vi "FlexMag - 23-03-2023.vi"() -> ()   [LabVIEW 2018]
uses:
  <vilib>/Instr/_visa.llb/VISA Configure Serial Port (Instr).vi
  nimodbus121/71/vi.lib/NI Modbus.llb/MB Serial Master Query Write Single Coil (poly).vi
  <vilib>/picture/picture.llb/Draw True-Color Pixmap.vi
  <vilib>/Utility/file.llb/Read Delimited Spreadsheet (string).vi
  <vilib>/addons/control/pid/pid.llb/PID (DBL).vi
  <vilib>/addons/control/pid/NI_PID_pid.lvlib
panel:
  in  "initial cover tab":enum32{"Page 1"}(tab)
  out "initial string":string
  out "Slide":u8(slide) scale=0.0..100.0
  out "MAG gui":bool
  in  "buzzer off":bool
  in  "ABORT":bool
  out "Description":string
  out "Warning Message":string
  in  "clear warning":bool
  out "System Status":string
  in  "Recipe Tab":enum32{"Page 1", "Page 2", "Page 3"}(tab)
  in  "R Recipe Selection":u16(ring) items=["single recipe", "multilayer recipe"]
  in  "R Web Selection":u16(ring) items=["web", "other"]
  in  "R tension value":dbl=8.0
  in  "R web speed":dbl=250.0
  in  "R web thickness":dbl=50.0
  in  "R left initial diameter":dbl
  in  "R core diameter":dbl=93.0
  in  "R Ar set sccm":dbl=20.0
  in  "R Pressure set mbar":dbl=0.005 format="%#_1e"
  in  "R DC Sputter Chamber Selection":enum32{"chamber II", "chamber III"}(radio)
  in  "R single process selection":enum32{"microwave", "dcsputter", "rfsputter"}(radio)
  in  "R Substrate Material":string
  in  "R Recipe Name":string
  in  "load recipe from path":bool
  out "path for loading recipe":path
  out "process file list 2":string
  out "L dc step numbers":string
  out "L rf step numbers":string
  out "L pressure":string
  out "L argon flow":string
  out "L rf length step 10":string
  out "L rf length step 9":string
  out "L rf length step 8":string
  out "L rf length step 7":string
  out "L rf length step 6":string
  out "L rf length step 5":string
  out "L rf length step 4":string
  out "L rf length step 3":string
  out "L rf length step 2":string
  out "L rf length step 1":string
  out "L rf power step 10":string
  out "L rf power step 9":string
  out "L rf power step 8":string
  out "L rf power step 7":string
  out "L rf power step 6":string
  out "L rf power step 5":string
  out "L rf power step 4":string
  out "L rf power step 3":string
  out "L rf power step 2":string
  out "L rf power step 1":string
  out "L dc length step 10":string
  out "L dc length step 9":string
  out "L dc length step 8":string
  out "L dc length step 7":string
  out "L dc length step 6":string
  out "L dc length step 5":string
  out "L dc length step 4":string
  out "L dc length step 3":string
  out "L dc length step 2":string
  out "L dc length step 1":string
  out "L dc power step 10":string
  out "L dc power step 9":string
  out "L dc power step 8":string
  out "L dc power step 7":string
  out "L dc power step 6":string
  out "L dc power step 5":string
  out "L dc power step 4":string
  out "L dc power step 3":string
  out "L dc power step 2":string
  out "L dc power step 1":string
  out "L microwave power":string
  out "L chamber selection":string
  out "L single process type selection":string
  out "L tension  value":string
  out "L web speed":string
  out "L web thickness":string
  out "L left init diamater":string
  out "L core diamater":string
  out "L web selection":string
  out "L recipe selection":string
  out "L sbs name":string
  out "L recipe name":string
  out "L dc power step 11":string
  out "L dc power step 12":string
  out "L dc power step 13":string
  out "L dc power step 14":string
  out "L dc power step 15":string
  out "L dc power step 16":string
  out "L dc power step 17":string
  out "L dc power step 18":string
  out "L dc power step 19":string
  out "L dc power step 20":string
  out "L dc length step 11":string
  out "L dc length step 12":string
  out "L dc length step 13":string
  out "L dc length step 14":string
  out "L dc length step 15":string
  out "L dc length step 16":string
  out "L dc length step 17":string
  out "L dc length step 18":string
  out "L dc length step 19":string
  out "L dc length step 20":string
  out "L rf power step 11":string
  out "L rf power step 12":string
  out "L rf power step 13":string
  out "L rf power step 14":string
  out "L rf power step 15":string
  out "L rf power step 16":string
  out "L rf power step 17":string
  out "L rf power step 18":string
  out "L rf power step 19":string
  out "L rf power step 20":string
  out "L rf length step 11":string
  out "L rf length step 12":string
  out "L rf length step 13":string
  out "L rf length step 14":string
  out "L rf length step 15":string
  out "L rf length step 16":string
  out "L rf length step 17":string
  out "L rf length step 18":string
  out "L rf length step 19":string
  out "L rf length step 20":string
  in  "R DC number steps":dbl
  in  "R rf step length 1":dbl
  in  "R rf step length 2":dbl
  in  "R rf step length 3":dbl
  in  "R rf step length 4":dbl
  in  "R rf step length 6":dbl
  in  "R rf step length 7":dbl
  in  "R rf step length 8":dbl
  in  "R rf step length 9":dbl
  in  "R rf step length 5":dbl
  in  "R rf step length 10":dbl
  in  "R dc step power 1":dbl
  in  "R dc step power 2":dbl
  in  "R dc step power 3":dbl
  in  "R dc step power 4":dbl
  in  "R dc step power 6":dbl
  in  "R dc step power 7":dbl
  in  "R dc step power 8":dbl
  in  "R dc step power 9":dbl
  in  "R dc step power 5":dbl
  in  "R dc step power 10":dbl
  in  "R dc step length 1":dbl
  in  "R dc step length 2":dbl
  in  "R dc step length 3":dbl
  in  "R dc step length 4":dbl
  in  "R dc step length 6":dbl
  in  "R dc step length 7":dbl
  in  "R dc step length 8":dbl
  in  "R dc step length 9":dbl
  in  "R dc step length 5":dbl
  in  "R dc step length 10":dbl
  in  "R rf step power 1":dbl
  in  "R rf step power 2":dbl
  in  "R rf step power 3":dbl
  in  "R rf step power 4":dbl
  in  "R rf step power 8":dbl
  in  "R rf step power 5":dbl
  in  "R rf step power 6":dbl
  in  "R rf step power 9":dbl
  in  "R rf step power 7":dbl
  in  "R rf step power 10":dbl
  in  "R power microwave":dbl
  in  "R RF number steps":dbl
  in  "R dc step power 11":dbl
  in  "R dc step power 12":dbl
  in  "R dc step power 13":dbl
  in  "R dc step power 14":dbl
  in  "R dc step power 15":dbl
  in  "R dc step power 16":dbl
  in  "R dc step power 17":dbl
  in  "R dc step power 18":dbl
  in  "R dc step power 19":dbl
  in  "R dc step power 20":dbl
  in  "R dc step length 11":dbl
  in  "R dc step length 12":dbl
  in  "R dc step length 13":dbl
  in  "R dc step length 14":dbl
  in  "R dc step length 15":dbl
  in  "R dc step length 16":dbl
  in  "R dc step length 17":dbl
  in  "R dc step length 18":dbl
  in  "R dc step length 19":dbl
  in  "R dc step length 20":dbl
  in  "GUI_Tab":T1(tab)
  in  "Tab Pressure Graph":enum32{"CH 1", "CH 2", "CH 3", "CH 4"}(tab)
  out "CH 1 Pressure":dbl(graph)
  out "CH 2 Pressure":dbl(graph)
  out "CH 3 Pressure":dbl(graph)
  out "CH 4 Pressure":dbl(graph)
  in  "pid graph":enum32{"Page 1"}(tab)
  out "Waveform Chart":dbl(graph)
  in  "cc3 timer tab":enum32{"Page 1"}(tab)
  in  "cc3 open gui":bool
  in  "cc3 close gui":bool
  in  "cc1 timer tab":enum32{"Page 1"}(tab)
  in  "cc1 close gui":bool
  in  "cc1 open gui":bool
  in  "cc2 timer tab":enum32{"Page 1"}(tab)
  in  "cc2 open gui":bool
  in  "cc2 close gui":bool
  in  "cc4 timer tab":enum32{"Page 1"}(tab)
  in  "cc4 open gui":bool
  in  "cc4 close gui":bool
  in  "bgbv2 timer tab":enum32{"Page 1"}(tab)
  in  "bgbv2 open gui":bool
  in  "bgbv2 close gui":bool
  in  "bgbv3 timer tab":enum32{"Page 1"}(tab)
  in  "bgbv3 open gui":bool
  in  "bgbv3 close gui":bool
  in  "bgbv1 timer tab":enum32{"Page 1"}(tab)
  in  "bgbv1 close gui":bool
  in  "bgbv1 open gui":bool
  in  "bgbv4 timer tab":enum32{"Page 1"}(tab)
  in  "bgbv4 open gui":bool
  in  "bgbv4 close gui":bool
  in  "tp1 timer tab":enum32{"Page 1"}(tab)
  in  "Tp1 stop gui":bool
  in  "Tp1 start gui":bool
  out "ch1_2 vacuum level":string
  out "ch2_3 vacuum level":string
  out "ch3_4 vacuum level":string
  in  "CH3-4 trnsgv timer tab":enum32{"Page 1"}(tab)
  in  "CH3-4 trns open gui":bool
  in  "CH3-4 trns close gui":bool
  in  "CH2-3 trnsgv timer tab":enum32{"Page 1"}(tab)
  in  "CH2-3 trns open gui":bool
  in  "CH2-3 trns close gui":bool
  in  "CH1-2 trnsgv timer tab":enum32{"Page 1"}(tab)
  in  "CH1-2 trns open gui":bool
  in  "CH1-2 trns close gui":bool
  in  "ch4 trnsbp right timer tab":enum32{"Page 1"}(tab)
  in  "ch4 trnsbp right close gui":bool
  in  "ch4 trnsbp right open gui":bool
  in  "ch3 trnsbp left timer tab":enum32{"Page 1"}(tab)
  in  "ch3 trnsbp left close gui":bool
  in  "ch3 trnsbp left open gui":bool
  in  "ch3 trnsbp right timer tab":enum32{"Page 1"}(tab)
  in  "ch3 trnsbp right close gui":bool
  in  "ch3 trnsbp right open gui":bool
  in  "ch2 trnsbp left timer tab":enum32{"Page 1"}(tab)
  in  "ch2 trnsbp left close gui":bool
  in  "ch2 trnsbp left open gui":bool
  in  "ch2 trnsbp right timer tab":enum32{"Page 1"}(tab)
  in  "ch2 trnsbp right close gui":bool
  in  "ch2 trnsbp right open gui":bool
  in  "ch1 trnsbp left timer tab":enum32{"Page 1"}(tab)
  in  "ch1 trnsbp left close gui":bool
  in  "ch1 trnsbp left open gui":bool
  out "ch4 ch pg mbar gui":dbl format="%#_2e"
  out "ch4 cc mbar gui":dbl format="%#_2e"
  out "ch4 pl pg mbar gui":dbl format="%#_2e"
  out "ch3 cc mbar gui":dbl format="%#_2e"
  out "ch3 ch pg mbar gui":dbl format="%#_2e"
  out "ch3 pl pg mbar gui":dbl format="%#_2e"
  out "ch2 ch pg mbar gui":dbl format="%#_2e"
  out "ch2 pl pg mbar gui":dbl format="%#_2e"
  out "ch2 cc mbar gui":dbl format="%#_2e"
  out "ch1 cc mbar gui":dbl format="%#_2e"
  out "ch1 ch pg mbar gui":dbl format="%#_2e"
  out "ch1 pl pg mbar gui":dbl format="%#_2e"
  out "Tp1 speed gui":i32
  out "Tp2 speed gui":i32
  out "Tp3 speed gui":i32
  out "Tp4 speed gui":i32
  in  "tp3 timer tab":enum32{"Page 1"}(tab)
  in  "Tp3 stop gui":bool
  in  "Tp3 start gui":bool
  in  "tp4 timer tab":enum32{"Page 1"}(tab)
  in  "Tp4 stop gui":bool
  in  "Tp4 start gui":bool
  in  "tp2 timer tab":enum32{"Page 1"}(tab)
  in  "Tp2 stop gui":bool
  in  "Tp2 start gui":bool
  in  "pcgv4 timer tab":enum32{"Page 1"}(tab)
  in  "pcgv4 open gui":bool
  in  "pcgv4 close gui":bool
  in  "pcgv3 timer tab":enum32{"Page 1"}(tab)
  in  "pcgv3 close gui":bool
  in  "pcgv3 open gui":bool
  in  "pcgv2 timer tab":enum32{"Page 1"}(tab)
  in  "pcgv2 close gui":bool
  in  "pcgv2 open gui":bool
  in  "pcgv1 timer tab":enum32{"Page 1"}(tab)
  in  "pcgv1 close gui":bool
  in  "pcgv1 open gui":bool
  out "Ch1_baratron_pressure_mbar":dbl format="%.1e"
  out "Ch2_baratron_pressure_mbar":dbl format="%.1e"
  out "Ch3_baratron_pressure_mbar":dbl format="%.1e"
  out "Ch4_baratron_pressure_mbar":dbl format="%.1e"
  in  "tpbv3 timer tab":enum32{"Page 1"}(tab)
  in  "tpbv3 open gui":bool
  in  "tpbv3 close gui":bool
  in  "tpbv2 timer tab":enum32{"Page 1"}(tab)
  in  "tpbv2 open gui":bool
  in  "tpbv2 close gui":bool
  in  "tpbv1 timer tab":enum32{"Page 1"}(tab)
  in  "tpbv1 close gui":bool
  in  "tpbv1 open gui":bool
  in  "chvbv4 timer tab":enum32{"Page 1"}(tab)
  in  "chvbv4 open gui":bool
  in  "chvbv4 close gui":bool
  in  "chvbv3 timer tab":enum32{"Page 1"}(tab)
  in  "chvbv3 open gui":bool
  in  "chvbv3 close gui":bool
  in  "chvbv2 timer tab":enum32{"Page 1"}(tab)
  in  "chvbv2 open gui":bool
  in  "chvbv2 close gui":bool
  in  "chvbv1 timer tab":enum32{"Page 1"}(tab)
  in  "chvbv1 close gui":bool
  in  "chvbv1 open gui":bool
  in  "tpbv4 timer tab":enum32{"Page 1"}(tab)
  in  "tpbv4 open gui":bool
  in  "tpbv4 close gui":bool
  in  "plvbv4 timer tab":enum32{"Page 1"}(tab)
  in  "plvbv4 open gui":bool
  in  "plvbv4 close gui":bool
  in  "plvbv3 timer tab":enum32{"Page 1"}(tab)
  in  "plvbv3 open gui":bool
  in  "plvbv3 close gui":bool
  in  "plvbv1 timer tab":enum32{"Page 1"}(tab)
  in  "plvbv1 close gui":bool
  in  "plvbv1 open gui":bool
  in  "plvbv2 timer tab":enum32{"Page 1"}(tab)
  in  "plvbv2 open gui":bool
  in  "plvbv2 close gui":bool
  in  "mp4 timer tab":enum32{"Page 1"}(tab)
  in  "mp4 start gui":bool
  in  "mp4 stop gui":bool
  in  "mp3 timer tab":enum32{"Page 1"}(tab)
  in  "mp3 start gui":bool
  in  "mp3 stop gui":bool
  in  "mp2 timer tab":enum32{"Page 1"}(tab)
  in  "mp2 start gui":bool
  in  "mp2 stop gui":bool
  in  "mp1 timer tab":enum32{"Page 1"}(tab)
  in  "mp1 start gui":bool
  in  "mp1 stop gui":bool
  in  "Tab Control":T2(tab)
  in  "OK Button":bool
  in  "cassette position selection":u16(ring)=1 items=["CH1"=1, "CH2"=2, "CH3"=3, "CH4"=4]
  in  "hide pressure graphs":bool
  in  "show pressure graphs":bool
  in  "graph sec":dbl=3.0
  in  "transfer vacuum":bool
  out "present location":dbl=inf format="%#_2g"
  in  "target chamber":dbl=1.0 min=1.0 max=4.0
  in  "transfer atm":bool
  in  "CHAMBERS CONTROL":T3(tab)
  in  "Tp1 normal speed gui":bool
  in  "Tp1 low speed gui":bool
  in  "Tp1 set speed gui":bool
  in  "Low_speed_value":ext=60.0
  in  "Pump Down CH1":bool
  in  "Shut Down CH1":bool
  in  "ch1 desired pressure":dbl format="%#_2e"
  in  "Low_speed_value 2":ext=60.0
  in  "Tp2 normal speed gui":bool
  in  "Tp2 low speed gui":bool
  in  "Tp2 set speed gui":bool
  in  "Pump Down CH2":bool
  in  "Shut Down CH2":bool
  in  "ch2 desired pressure":dbl format="%#_2e"
  in  "Low_speed_value 3":ext=60.0
  in  "Tp3 normal speed gui":bool
  in  "Tp3 low speed gui":bool
  in  "Tp3 set speed gui":bool
  in  "Pump Down CH3":bool
  in  "Shut Down CH3":bool
  in  "ch3 desired pressure":dbl format="%#_2e"
  in  "Pump Down CH4":bool
  in  "Shut Down CH4":bool
  in  "ch4 desired pressure":dbl=5e-05 format="%#_2e"
  in  "Low_speed_value 4":ext=60.0
  in  "Tp4 normal speed gui":bool
  in  "Tp4 low speed gui":bool
  in  "Tp4 set speed gui":bool
  in  "QR continuous mode gui":bool
  in  "QR off mode gui":bool
  out "qr read statue gui":string
  in  "max rotation number":dbl=300.0
  out "current step":dbl
  in  "step count":dbl
  out "lap number left actual":dbl
  out "lap number right actual":dbl
  in  "tension value":dbl=10.0
  in  "setpoint":dbl=550.0
  out "process variable":dbl
  out "ch4_srv_piston_status":string
  out "ch3_srv_piston_status":string
  out "ch2_srv_piston_status":string
  out "ch1_srv_piston_status":string
  out "ch4_petcool_status":string
  out "ch3_petcool_status":string
  out "ch2_petcool_status":string
  out "ch1_petcool_status":string
  out "ch4_cst_fix_status":string
  out "ch3_cst_fix_status":string
  out "ch2_cst_fix_status":string
  out "ch1_cst_fix_status":string
  in  "forward roll":bool
  in  "back roll":bool
  in  "stop roll":bool
  out "parameters led":bool
  in  "CH1 cstfix up":bool
  in  "CH1 cstfix down":bool
  in  "CH2 cstfix down":bool
  in  "CH2 cstfix up":bool
  in  "CH4 cstfix down":bool
  in  "CH4 cstfix up":bool
  in  "CH3 cstfix down":bool
  in  "CH3 cstfix up":bool
  in  "CH1 petcool down":bool
  in  "CH1 petcool up":bool
  in  "CH2 petcool down":bool
  in  "CH2 petcool up":bool
  in  "CH3 petcool down":bool
  in  "CH3 petcool up":bool
  in  "CH4 petcool down":bool
  in  "CH4 petcool up":bool
  in  "CH4 srv back":bool
  in  "CH4 srv forward":bool
  in  "CH3 srv back":bool
  in  "CH3 srv forward":bool
  in  "CH2 srv back":bool
  in  "CH2 srv forward":bool
  in  "CH1 srv back":bool
  in  "CH1 srv forward":bool
  in  "cycle roll stop":bool
  in  "cycle roll start":bool
  out "Remaining Cycle":u8
  in  "Number of Cycle":u8=10 min=1
  out "rolling direction gui":bool
  in  "load process file":bool
  in  "stop coating":bool
  in  "coating start":bool
  in  "CH1 LN2":bool
  in  "Stop auto LN2":bool
  in  "CH4 LN2":bool
  in  "CH2 LN2":bool
  in  "CH3 LN2":bool
  in  "water bypass":bool=TRUE
  out "process file list":string
  out "current recipe number":i32
  in  "creat recipe file":bool
  in  "creat process file":bool
  in  "Change Rolling Direction":bool
  out "Total Status":string
  out "Total Warning":string
  in  "hide service tab":bool
  in  "show service tab":bool
  in  "service tab":string
  out "ch1_door_open":string
  out "ch2_door_open":string
  out "ch4_door_open":string
  out "ch3_door_open":string
  out "General View":picture
  in  "bgbv4 close gui 2":bool
  in  "bgbv4 open gui 2":bool
  in  "sov4 timer tab":enum32{"Page 1"}(tab)
  in  "sov4 close gui":bool
  in  "sov4 open gui":bool
  out "ch4 ch pg mbar gui 1":dbl format="%#_2e"
  out "ch4 cc mbar gui 1":dbl format="%#_2e"
  out "Ch4_baratron_pressure_mbar 2":dbl format="%.1e"
  out "CH4 front main":picture
  out "CH4 top main":picture
  in  "cc4 close gui 2":bool
  in  "cc4 open gui 2":bool
  in  "Baratron4 set zero gui":bool
  in  "pcgv4 set pressure":bool
  in  "pcgv4 set position gui":bool
  out "pcgv4 position":i32
  in  "pcgv4 set position value":dbl
  in  "pcgv4 set pressure value mbar":dbl=0.005 format="%.1e"
  in  "sov4 close gui 2":bool
  in  "sov4 open gui 2":bool
  out "Ch4_baratron_pressure_mbar 3":dbl format="%.1e"
  in  "Rf_control_tab":T4(tab)
  in  "RF off":bool
  in  "RF on":bool
  in  "RF host":bool
  out "RF Net Power :":u32
  in  "set rf":bool
  in  "RF_forward_power_1":i16
  out "RF Bias:":u32
  in  "Ramp up Time:":dbl
  out "Ramp Up Left Time:":dbl
  in  "Ramp Down Time :":dbl
  out "Ramp Down Left Time:":dbl
  in  "Ramp Up time":bool
  in  "Ramp down time":bool
  out "Pulsing ON/OFF :":bool
  in  "Duty Cycle :":i8
  in  "Frequency :":i64 caption="FREQUENCY"
  in  "set frequency":bool
  in  "set duty":bool
  in  "Pulsing_off":bool
  in  "internal":bool
  in  "Set CL Position:":dbl
  in  "Set CT Position:":dbl
  out "CL Position:":dbl
  out "CT Position:":dbl
  in  "set seri cap pos 2":bool
  in  "set cap pos":bool
  in  "oto tuner":bool
  in  "manuel tuner":bool
  in  "ch4 ar set zero":bool
  in  "ch4 ar set":bool
  out "ch4 argon mfc actual":dbl format="%#.3f"
  in  "ch4 argon mfc set":dbl
  in  "CH3 water close gui":bool
  in  "CH3 water open gui":bool
  in  "bgbv3 open gui 2":bool
  in  "bgbv3 close gui 2":bool
  out "CH3 MAG Active":bool
  in  "ch3 mag active gui":bool
  in  "sov3 timer tab":enum32{"Page 1"}(tab)
  in  "sov3 close gui":bool
  in  "sov3 open gui":bool
  out "ch3 cc mbar gui 1":dbl format="%#_2e"
  out "ch3 ch pg mbar gui 1":dbl format="%#_2e"
  out "Ch3_baratron_pressure_mbar 2":dbl format="%.1e"
  out "CH3 front main":picture
  out "CH3 top main":picture
  in  "cc3 open gui 2":bool
  in  "cc3 close gui 2":bool
  in  "Baratron3 auto set zero":bool
  in  "pcgv3 set pressure gui":bool
  in  "pcgv3 set position":bool
  out "pcgv3 position":i32
  in  "pcgv3 set position value":dbl
  in  "pcgv3 set pressure value mbar":dbl=0.005 format="%.1e"
  in  "sov3 open gui 2":bool
  in  "sov3 close gui 2":bool
  out "Ch3_baratron_pressure_mbar 3":dbl format="%.1e"
  in  "ch3 argon mfc set":dbl
  out "ch3 argon mfc actual":dbl format="%#.3f"
  in  "ch3 ar set":bool
  in  "ch3 ar set zero":bool
  in  "DC_ramp_down 2":bool
  in  "DC_ramp_up 2":bool
  in  "Dc_set_zero 2":bool
  in  "Dc_set_ch3":bool
  in  "Dc_off_2":bool
  in  "Dc_on_2":bool
  in  "DC_host 2":bool
  out "Actual DC Power : 2":dbl format="%#.0f"
  out "Actual DC Volt2":dbl format="%#.0f"
  in  "Set DC Power ch3":dbl
  in  "DC_ramp_up_time : 2":dbl
  in  "DC_ramp_down_time: 2":dbl
  in  "CH2 water close gui":bool
  in  "CH2 water open gui":bool
  in  "bgbv2 close gui 2":bool
  in  "bgbv2 open gui 2":bool
  out "CH2 MAG Active":bool
  in  "ch2 mag active gui":bool
  in  "sov2 timer tab":enum32{"Page 1"}(tab)
  in  "sov2 close gui":bool
  in  "sov2 open gui":bool
  out "ch2 ch pg mbar gui 1":dbl format="%#_2e"
  out "ch2 cc mbar gui 1":dbl format="%#_2e"
  out "Ch2_baratron_pressure_mbar 2":dbl format="%.1e"
  out "CH2 front main":picture
  out "CH2 top main":picture
  in  "cc2 close gui 2":bool
  in  "cc2 open gui 2":bool
  in  "Baratron2 set zero gui":bool
  in  "pcgv2 set pressure gui":bool
  in  "pcgv2 set position gui":bool
  out "pcgv2 position":i32
  in  "pcgv2 set position value":dbl
  in  "pcgv2 set pressure value mbar":dbl=0.005 format="%.1e"
  in  "sov2 open gui 2":bool
  in  "sov2 close gui 2":bool
  out "Ch2_baratron_pressure_mbar 3":dbl format="%.1e"
  in  "ch2 argon mfc set":dbl
  in  "ch2 ar set zero":bool
  out "ch2 argon mfc actual":dbl format="%#.3f"
  in  "ch2 ar set":bool
  in  "Dc_set_ch2":bool
  in  "Dc_off":bool
  in  "Dc_on":bool
  in  "Dc_set_zero":bool
  in  "DC_ramp_up_time :":dbl
  in  "DC_ramp_down_time:":dbl
  in  "Set DC Power ch2":dbl
  out "Actual DC Power":dbl format="%#.0f"
  in  "DC_ramp_down":bool
  in  "DC_ramp_up":bool
  out "Actual DC Volt :":dbl format="%#.0f"
  in  "DC_host":bool
  in  "bgbv1 close gui 2":bool
  in  "bgbv1 open gui 2":bool
  in  "Baratron1 set zero gui":bool
  in  "pcgv1 set pressure gui":bool
  in  "pcgv1 set position":bool
  out "pcgv1 position":i32
  in  "pcgv1 set position value":dbl
  in  "pcgv1 set pressure value mbar":dbl=0.005 format="%.1e"
  out "Ch1_baratron_pressure_mbar 3":dbl format="%.1e"
  in  "sov1 close gui 2":bool
  in  "sov1 open gui 2":bool
  in  "sov1 timer tab":enum32{"Page 1"}(tab)
  in  "sov1 close gui":bool
  in  "sov1 open gui":bool
  out "ch1 ch pg mbar gui 1":dbl format="%#_2e"
  out "ch1 cc mbar gui 1":dbl format="%#_2e"
  out "Ch1_baratron_pressure_mbar 2":dbl format="%.1e"
  out "CH1 front main":picture
  out "CH1 top main":picture
  in  "cc1 close gui 2":bool
  in  "cc1 open gui 2":bool
  in  "MWPS1 close":bool
  in  "MWPS1 open":bool
  in  "MWPS1 set":dbl
  in  "MWPS2 close":bool
  in  "MWPS2 open":bool
  in  "MWPS2 set":dbl
  in  "ch1 ar set":bool
  in  "ch1 ar set zero":bool
  out "ch1 argon mfc actual":dbl format="%#.3f"
  in  "ch1 argon mfc set":dbl
  in  "Technical Service":T5(tab)
  out "Interrupt DI":bool=TRUE
  in  "Center MOXA":enum32{"DI/DO 1", "DI/DO 2", "AO/AI"}(tab)
  in  "Casette_Servo_Start/Stop DO":bool
  in  "Casette_Servo_Left_Direction DO":bool
  in  "Tension_Controllers_Start/Stop DO":bool
  in  "Cnt_Right_Limit DO":bool
  in  "Cnt_Left_Limit DO":bool
  in  "Cnt_Right_Slow DO":bool
  in  "Cnt_Left_Slow DO":bool
  in  "Buzzer DO":bool
  out "Casette_Servo_Start/Stop DI":bool
  out "Casette_Servo_Left_Direction DI":bool
  out "Cnt_Right_Limit DI":bool
  out "Tension_Controllers_Start/Stop DI":bool
  out "WFC DI":bool
  out "Cnt_Left_Limit DI":bool
  out "Cnt_Left_Slow DI":bool
  out "Cnt_Right_Slow DI":bool
  in  "Center_2 DO8":bool
  in  "Center_2 DO6":bool
  in  "Center_2 DO5":bool
  in  "Center_2 DO7":bool
  in  "DCPS_ SW4 DO":bool
  in  "DCPS_ SW3  DO":bool
  in  "DCPS_ SW2 DO":bool
  in  "DCPS_ SW1 DO":bool
  out "Center_2 DI8":bool
  out "Center_2 DI7":bool
  out "MW2 DI":bool
  out "MW1 DI":bool
  out "DCPS_ SW4 DI":bool
  out "DCPS_ SW3 DI":bool
  out "DCPS_ SW2 DI":bool
  out "DCPS_ SW1 DI":bool
  in  "TC2 Set moxa":bool
  in  "TC1 Set moxa":bool
  in  "Cassette_Servo_Speed Set":bool
  in  "TC2_Set_Value_Moxa":dbl
  in  "TC1_Set_Value_Moxa":dbl
  in  "Cassette_Servo_Speed AO":dbl
  in  "Center AO1":dbl
  in  "Center AO1 Set":bool
  in  "CH1_Motor DO":bool
  in  "CH2_Motor DO":bool
  in  "CH4_Motor DO":bool
  in  "CH3_Motor DO":bool
  out "Ch1_srv1_counter DI":bool
  out "Ch2_srv1_counter DI":bool
  out "Ch4_srv1_counter DI":bool
  out "Ch3_srv1_counter DI":bool
  out "Center_4 DI7":bool
  out "Center_4 DI6":bool
  out "Center_4 DI5":bool
  out "element":bool
  in  "CH1 MOXA":T6(tab)
  in  "CH1_CC_DO":bool
  in  "CH1_PL_VBV_DO":bool
  in  "CH1_CH_ATM_DO":bool
  in  "CH1_PL_ATM_DO":bool
  in  "CH1_CH_VBV_DO":bool
  in  "CH1_BG_BV_DO":bool
  in  "CH1_TP_BV_DO":bool
  in  "CH1_MP_DO":bool
  out "CH1_CC_DI":bool
  out "CH1_PL_ATM_DI":bool
  out "CH1_PL_VBV_DI":bool
  out "CH1_CH_ATM_DI":bool
  out "CH1_CH_VBV_DI":bool
  out "CH1_BG_BV_DI":bool
  out "CH1_TP_BV_DI":bool
  out "CH1_MP_DI":bool
  in  "CH1_PetCool_Down_DO":bool
  in  "CH1_M2_D6_DO":bool
  in  "CH1_Cst_Fix_DO":bool
  in  "CH1_PetCool_Up_DO":bool
  in  "CH1_M2_D4_DO":bool
  in  "CH1_Trns_Gv_Close_DO":bool
  in  "CH1_Trns_Gv_Open_DO":bool
  in  "CH1_SoV_Ar_DO":bool
  out "CH1_PetCool_Down_DI":bool
  out "CH1_PetCool_Up_DI":bool
  out "CH1_Cst_Fix_Down_DI":bool
  out "CH1_Cst_Fix_Up_DI":bool
  out "CH1_M2_D4_DI":bool
  out "CH1_Trns_Gv_Close_DI":bool
  out "CH1_Trns_Gv_Open_DI":bool
  out "CH1_SoV_Ar_DI":bool
  in  "CH1_Trns_BP_Left_DO":bool
  in  "CH1_M3_D6_DO":bool
  in  "CH1_M3_D5_DO":bool
  in  "CH1_WFC_DO":bool
  in  "CH1_SRV_Direction_Clockwise_DO":bool
  in  "CH1_M3_D3_DO":bool
  in  "CH1_SRV1_Piston_Back_DO":bool
  in  "CH1_SRV1_Piston_For_DO":bool
  out "CH1_Trns_BP_Left_DI":bool
  out "CH1_WFC_DI":bool
  out "CH1_M3_D6_DI":bool
  out "CH1_SRV2_COUNTER_DI":bool
  out "CH1_SRV_Left_Direction_DI":bool
  out "CH1_SRV_Start_Stop_DI":bool
  out "CH1_SRV1_Piston_Back_DI":bool
  out "CH1_SRV1_Piston_For_DI":bool
  in  "CH1_M4_D8_DO":bool
  in  "CH1_Right_Slow_DO":bool
  in  "CH1_Right_Limit_DO":bool
  in  "CH1_M4_D7_DO":bool
  in  "CH1_M4_D4_DO":bool
  in  "CH1_TGV_Control_DO":bool
  in  "CH1_M4_D2_DO":bool
  in  "CH1_LN2_DO":bool
  out "CH1_M4_D8_DI":bool
  out "CH1_M4_D7_DI":bool
  out "CH1_Right_Slow_DI":bool
  out "CH1_Right_Limit_DI":bool
  out "CH1_Trns_Interlock_DI":bool
  out "CH1_TGV_Control_DI":bool
  out "CH1_DS_DI":bool
  out "CH1_Air_Pressure_DI":bool
  out "CH1_Ai_A4":u16
  out "CH1_Ai_Ch_Cc":u16
  out "CH1_LN2_TK_b":u16
  out "CH1_LN2_TK_t":u16
  out "CH1_Ai_A6":u16
  out "CH1_Ai_A5":u16
  out "CH1_Ai_Ch_Pg":u16
  out "CH1_Ai_Pl_Pg":u16
  in  "CH1 AO3 Set":bool
  in  "CH1 AO4 Set":bool
  in  "CH1 MW2 Set":bool
  in  "CH1 MW1 Set":bool
  in  "CH1 MW1":dbl
  in  "CH1 MW2":dbl
  in  "CH1 AO3":dbl
  in  "CH1 AO4":dbl
  in  "CH2 MOXA":T6(tab)
  in  "CH2_CC_DO":bool
  in  "CH2_PL_VBV_DO":bool
  in  "CH2_CH_ATM_DO":bool
  in  "CH2_PL_ATM_DO":bool
  in  "CH2_CH_VBV_DO":bool
  in  "CH2_BG_BV_DO":bool
  in  "CH2_TP_BV_DO":bool
  in  "CH2_MP_DO":bool
  out "CH2_CC_DI":bool
  out "CH2_PL_ATM_DI":bool
  out "CH2_PL_VBV_DI":bool
  out "CH2_CH_ATM_DI":bool
  out "CH2_CH_VBV_DI":bool
  out "CH2_BG_BV_DI":bool
  out "CH2_TP_BV_DI":bool
  out "CH2_MP_DI":bool
  in  "CH2_PetCool_Down_DO":bool
  in  "CH2_M2_D6_DO":bool
  in  "CH2_Cst_Fix_DO":bool
  in  "CH2_PetCool_Up_DO":bool
  in  "CH2_Trns_BP_Right_DO":bool
  in  "CH2_Trns_GV_Close_DO":bool
  in  "CH2_Trns_GV_Open_DO":bool
  in  "CH2_SoV_Ar_DO":bool
  out "CH2_PetCool_Down_DI":bool
  out "CH2_PetCool_Up_DI":bool
  out "CH2_Cst_Fix_Down_DI":bool
  out "CH2_Cst_Fix_Up_DI":bool
  out "CH2_Trns_BP_Right_DI":bool
  out "CH2_Trns_Gv_Close_DI":bool
  out "CH2_Trns_Gv_Open_DI":bool
  out "CH2_SoV_Ar_DI":bool
  in  "CH2_Trns_BP_Left_DO":bool
  in  "CH2_M3_D6_DO":bool
  in  "CH2_M3_D5_DO":bool
  in  "CH2_WFC_DO":bool
  in  "CH2_SRV_Direction_Clockwise_DO":bool
  in  "CH2_M3_D3_DO":bool
  in  "CH2_SRV1_Piston_Back_DO":bool
  in  "CH2_SRV1_Piston_For_DO":bool
  out "CH2_Trns_BP_Left_DI":bool
  out "CH2_WFC_DI":bool
  out "CH2_M3_D6_DI":bool
  out "CH2_SRV2_COUNTER_DI":bool
  out "CH2_SRV_Left_Direction_DI":bool
  out "CH2_SRV_Start_Stop_DI":bool
  out "CH2_SRV1_Piston_Back_DI":bool
  out "CH2_SRV1_Piston_For_DI":bool
  in  "CH2_Left_Limit_DO":bool
  in  "CH2_Right_Slow_DO":bool
  in  "CH2_Right_Limit_DO":bool
  in  "CH2_Left_Slow_DO":bool
  in  "CH2_M4_D4_DO":bool
  in  "CH2_TGV_Control_DO":bool
  in  "CH2_M4_D2_DO":bool
  in  "CH2_LN2_DO":bool
  out "CH2_Left_Limit_DI":bool
  out "CH2_Left_Slow_DI":bool
  out "CH2_Right_Slow_DI":bool
  out "CH2_Right_Limit_DI":bool
  out "CH2_Trns_Interlock_DI":bool
  out "CH2_TGV_Control_DI":bool
  out "CH2_DS_DI":bool
  out "CH2_Air_Pressure_DI":bool
  out "CH2_LN2_TK_b":u16
  out "CH2_LN2_TK_t":u16
  out "CH2_Ai_A6":u16
  out "CH2_Ai_A5":u16
  out "CH2_Ai_A4":u16
  out "CH2_Ai_Ch_Cc":u16
  out "CH2_Ai_Ch_Pg":u16
  out "CH2_Ai_Pl_Pg":u16
  in  "CH2 AO1":dbl
  in  "CH2 AO2":dbl
  in  "CH2 AO3":dbl
  in  "CH2 AO4":dbl
  in  "CH2 AO3 Set":bool
  in  "CH2 AO4 Set":bool
  in  "CH2 AO2 Set":bool
  in  "CH2 AO1 Set":bool
  in  "CH3 MOXA":T6(tab)
  in  "CH3_CC_DO":bool
  in  "CH3_PL_VBV_DO":bool
  in  "CH3_CH_ATM_DO":bool
  in  "CH3_PL_ATM_DO":bool
  in  "CH3_CH_VBV_DO":bool
  in  "CH3_BG_BV_DO":bool
  in  "CH3_TP_BV_DO":bool
  in  "CH3_MP_DO":bool
  out "CH3_CC_DI":bool
  out "CH3_PL_ATM_DI":bool
  out "CH3_PL_VBV_DI":bool
  out "CH3_CH_ATM_DI":bool
  out "CH3_CH_VBV_DI":bool
  out "CH3_BG_BV_DI":bool
  out "CH3_TP_BV_DI":bool
  out "CH3_MP_DI":bool
  in  "CH3_PetCool_Down_DO":bool
  in  "CH3_M2_D6_DO":bool
  in  "CH3_Cst_Fix_DO":bool
  in  "CH3_PetCool_Up_DO":bool
  in  "CH3_Trns_BP_Right_DO":bool
  in  "CH3_Trns_GV_Close_DO":bool
  in  "CH3_Trns_GV_Open_DO":bool
  in  "CH3_SoV_Ar_DO":bool
  out "CH3_PetCool_Down_DI":bool
  out "CH3_PetCool_Up_DI":bool
  out "CH3_Cst_Fix_Down_DI":bool
  out "CH3_Cst_Fix_Up_DI":bool
  out "CH3_Trns_BP_Right_DI":bool
  out "CH3_Trns_Gv_Close_DI":bool
  out "CH3_Trns_Gv_Open_DI":bool
  out "CH3_SoV_Ar_DI":bool
  in  "CH3_Trns_BP_Left_DO":bool
  in  "CH3_M3_D6_DO":bool
  in  "CH3_M3_D5_DO":bool
  in  "CH3_WFC_DO":bool
  in  "CH3_SRV_Direction_Clockwise_DO":bool
  in  "CH3_M3_D3_DO":bool
  in  "CH3_SRV1_Piston_Back_DO":bool
  in  "CH3_SRV1_Piston_For_DO":bool
  out "CH3_Trns_BP_Left_DI":bool
  out "CH3_WFC_DI":bool
  out "CH3_M3_D6_DI":bool
  out "CH3_SRV2_COUNTER_DI":bool
  out "CH3_SRV_Left_Direction_DI3":bool
  out "CH3_SRV_Start_Stop_DI":bool
  out "CH3_SRV1_Piston_Back_DI":bool
  out "CH3_SRV1_Piston_For_DI":bool
  in  "CH3_Left_Limit_DO":bool
  in  "CH3_Right_Slow_DO":bool
  in  "CH3_Right_Limit_DO":bool
  in  "CH3_Left_Slow_DO":bool
  in  "CH3_M4_D4_DO":bool
  in  "CH3_TGV_Control_DO":bool
  in  "CH3_M4_D2_DO":bool
  in  "CH3_LN2_DO":bool
  out "CH3_Left_Limit_DI":bool
  out "CH3_Left_Slow_DI":bool
  out "CH3_Right_Slow_DI":bool
  out "CH3_Right_Limit_DI":bool
  out "CH3_Trns_Interlock_DI":bool
  out "CH3_TGV_Control_DI":bool
  out "CH3_DS_DI":bool
  out "CH3_Air_Pressure_DI":bool
  out "CH3_LN2_TK_b":u16
  out "CH3_LN2_TK_t":u16
  out "CH3_Ai_A6":u16
  out "CH3_Ai_A5":u16
  out "MFC_Ar_Read_value":u16
  out "CH3_Ai_Ch_Cc":u16
  out "CH3_Ai_Ch_Pg":u16
  out "CH3_Ai_Pl_Pg":u16
  in  "CH3 AO3 Set":bool
  in  "MFC_Ar_Set":bool
  in  "CH3 AO2 Set":bool
  in  "CH3 AO1 Set":bool
  in  "CH3 AO1":dbl
  in  "CH3 AO2":dbl
  in  "CH3 AO3":dbl
  in  "MFC_Ar_Set_value":dbl
  in  "CH4 MOXA":T6(tab)
  in  "CH4_CC_DO":bool
  in  "CH4_PL_VBV_DO":bool
  in  "CH4_CH_ATM_DO":bool
  in  "CH4_PL_ATM_DO":bool
  in  "CH4_CH_VBV_DO":bool
  in  "CH4_BG_BV_DO":bool
  in  "CH4_TP_BV_DO":bool
  in  "CH4_MP_DO":bool
  out "CH4_CC_DI":bool
  out "CH4_PL_ATM_DI":bool
  out "CH4_PL_VBV_DI":bool
  out "CH4_CH_ATM_DI":bool
  out "CH4_CH_VBV_DI":bool
  out "CH4_BG_BV_DI":bool
  out "CH4_TP_BV_DI":bool
  out "CH4_MP_DI":bool
  in  "CH4_PetCool_Down_DO":bool
  in  "CH4_M2_D6_DO":bool
  in  "CH4_Cst_Fix_DO":bool
  in  "CH4_PetCool_Up_DO":bool
  in  "CH4_Trns_BP_Right_DO":bool
  in  "CH4_M2_D3_DO":bool
  in  "CH4_M2_D2_DO":bool
  in  "CH4_SoV_Ar_DO":bool
  out "CH4_PetCool_Down_DI":bool
  out "CH4_PetCool_Up_DI":bool
  out "CH4_Cst_Fix_Down_DI":bool
  out "CH4_Cst_Fix_Up_DI":bool
  out "CH4_Trns_BP_Right_DI":bool
  out "CH4_M2_D3_DI":bool
  out "CH4_M2_D2_DI":bool
  out "CH4_SoV_Ar_DI":bool
  in  "CH4_M3_D8_DO":bool
  in  "CH4_M3_D6_DO":bool
  in  "CH4_M3_D5_DO":bool
  in  "CH4_WFC_DO":bool
  in  "CH4_SRV_Direction_Clockwise_DO":bool
  in  "CH4_M3_D3_DO":bool
  in  "CH4_SRV1_Piston_Back_DO":bool
  in  "CH4_SRV1_Piston_For_DO":bool
  out "CH4_SRV1_Piston_For_DI":bool
  out "CH4_SRV1_Piston_Back_DI":bool
  out "CH4_SRV_Start_Stop_DI":bool
  out "CH4_SRV_Left_Direction_DI":bool
  out "CH4_SRV2_COUNTER_DI":bool
  out "CH4_M3_D6_DI":bool
  out "CH4_WFC_DI":bool
  out "CH4_M3_D8_DI":bool
  in  "CH4_Left_Limit_DO":bool
  in  "CH4_M4_D6_DO":bool
  in  "CH4_M4_D5_DO":bool
  in  "CH4_Left_Slow_DO":bool
  in  "CH4_M4_D4_DO":bool
  in  "CH4_TGV_Control_DO":bool
  in  "CH4_M4_D2_DO":bool
  in  "CH4_LN2_DO":bool
  out "CH4_Left_Limit_DI":bool
  out "CH4_Left_Slow_DI":bool
  out "CH4_M4_D6_DI":bool
  out "CH4_M4_D5_DI":bool
  out "CH4_Trns_Interlock_DI":bool
  out "CH4_TGV_Control_DI":bool
  out "CH4_DS_DI":bool
  out "CH4_Air_Pressure_DI":bool
  out "CH4_LN2_TK_b":u16
  out "CH4_LN2_TK_t":u16
  out "CH4_Ai_A6":u16
  out "CH4_Ai_A5":u16
  out "CH4_Ai_A4":u16
  out "CH4_Ai_Ch_Cc":u16
  out "CH4_Ai_Ch_Pg":u16
  out "CH4_Ai_Pl_Pg":u16
  in  "CH4 AO3 Set":bool
  in  "CH4 AO4 Set":bool
  in  "CH4 AO2 Set":bool
  in  "CH4 AO1 Set":bool
  in  "CH4 AO1":dbl
  in  "CH4 AO2":dbl
  in  "CH4 AO3":dbl
  in  "CH4 AO4":dbl
  in  "keysight port":refnum<visa-resource-name>="USB0::0x0957::0x1807::MY59080144::INSTR"
  in  "QR Scanner Com":refnum<visa-resource-name>="COM5"
  in  "Counter Com":refnum<visa-resource-name>="COM118"
  in  "RF Com":refnum<visa-resource-name>="COM125"
  in  "DCPS Com":refnum<visa-resource-name>="COM126"
  in  "TC2 Com":refnum<visa-resource-name>="COM99"
  in  "TC1 Com":refnum<visa-resource-name>="COM98"
  in  "Pfeiffer TP Com":refnum<visa-resource-name>="COM116"
  in  "Vat PC GV Com":refnum<visa-resource-name>="COM117"
  in  "CH4 I/O Com":refnum<visa-resource-name>="COM115"
  in  "CH3 I/O Com":refnum<visa-resource-name>="COM114"
  in  "CH2 I/O Com":refnum<visa-resource-name>="COM113"
  in  "CH1 I/O Com":refnum<visa-resource-name>="COM112"
  in  "Center I/O Com":refnum<visa-resource-name>="COM111"
  out "CH4 I/O Loading":bool
  out "CH3 I/O Loading":bool
  out "CH2 I/O Loading":bool
  out "CH1 I/O Loading":bool
  out "Center I/O Loading":bool
  in  "Center I I/O Com":refnum<visa-resource-name>="COM121"
  in  "Microwave1 Com":refnum<visa-resource-name>="COM101"
  in  "Microwave2 Com":refnum<visa-resource-name>="COM102"
  in  "power difference":dbl=50.0
  in  "dcps check active":bool
  in  "Set DC Power auto":dbl
  in  "Dc_host_auto":bool
  in  "Dc_auto_set_zero":bool
  in  "Dc_auto_set":bool
  in  "Dc_auto_ramp_down":bool
  in  "Dc_auto_off_ramp_up":bool
  in  "Dc_auto_on":bool
  in  "Dc_auto_off":bool
  in  "DC_auto_voltage_mode":bool
  in  "DC_auto_power_mode":bool
  in  "Dcps_fail":bool
  out "read buffer":string
  out "Dcps_is_on":bool
  in  "dcps check(sec)":dbl=14.0
  in  "RF_auto_on":bool
  in  "RF_auto_off":bool
  out "RF 1 On":bool
  out "Frequency":u32
  out "duty cycle":u32
  out "EXTERNAL PULSING":bool
  out "PULSING OFF":bool
  out "INTERNAL PULSING":bool
  out "DC BIAS REGULATION":bool
  out "LOAD  REGULATION":bool
  out "FORWARD   REGULATION":bool
  out "Forward Power":u32
  out "Reflected Power":u32
  out "x-y":u32
  in  "RF_auto_tuner":bool
  in  "Ramp Down time_auto":bool
  in  "RF_auto_set":bool
  in  "Ramp Up time_auto":bool
  in  "RF_auto_host":bool
  in  "external":bool
  in  "External":bool
  in  "Load":bool
  in  "Forward":bool
  in  "initialize":bool
  in  "microwave1 wait ms":u32=100
  out "microwave1 read":string
  in  "microwave2 wait ms":u32=100
  out "microwave2 read":string
  in  "MWPS1 auto close":bool
  in  "MWPS1 auto open":bool
  in  "MWPS2 auto close":bool
  in  "MWPS2 auto open":bool
  in  "baud rate (9600) 2":u32=9600
  in  "baud rate (9600) 1":u32=9600
  out "ch4 mp timer":bool
  out "ch3 mp timer":bool
  out "ch2 mp timer":bool
  out "ch1 mp timer":bool
  out "ch1 pl vbv timer":bool
  out "ch2 pl vbv timer":bool
  out "ch3 pl vbv timer":bool
  out "ch4 pl vbv timer":bool
  out "ch1 tp bv timer":bool
  out "ch2 tp bv timer":bool
  out "ch3 tp bv timer":bool
  out "ch4 tp bv timer":bool
  out "ch1 tp timer":bool
  out "ch2 tp timer":bool
  out "ch3 tp timer":bool
  out "ch4 tp timer":bool
  out "ch1 ch vbv timer":bool
  out "ch2 ch vbv timer":bool
  out "ch3 ch vbv timer":bool
  out "ch4 ch vbv timer":bool
  out "ch1 pc gv timer":bool
  out "ch2 pc gv timer":bool
  out "ch3 pc gv timer":bool
  out "ch4 pc gv timer":bool
  out "ch1 cc timer":bool
  out "ch2 cc timer":bool
  out "ch3 cc timer":bool
  out "ch4 cc timer":bool
  out "ch1 bg bv timer":bool
  out "ch2 bg bv timer":bool
  out "ch3 bg bv timer":bool
  out "ch4 bg bv timer":bool
  out "ch1-2 trns gv timer":bool
  out "ch2-3 trns gv timer":bool
  out "ch3-4 trns gv timer":bool
  out "ch2 trnsbp left timer":bool
  out "ch2 trnsbp right timer":bool
  out "ch1 trnsbp left timer":bool
  out "ch4 trnsbp right timer":bool
  out "ch3 trnsbp left timer":bool
  out "ch3 trnsbp right timer":bool
  in  "coating safety cancel":bool
  in  "dcps on safety":bool
  in  "trns safety cancel":bool
  in  "CH1 safety cancel":bool
  in  "ch3 mfc set safety":bool
  in  "ch4 mfc set safety":bool
  in  "ch1 mfc set safety":bool
  in  "ch2 mfc set safety":bool
  in  "sov3 open safety":bool
  in  "sov4 open safety":bool
  in  "sov1 open safety":bool
  in  "sov2 open safety":bool
  in  "bgbv3 open safety":bool
  in  "bgbv4 open safety":bool
  in  "bgbv1 open safety":bool
  in  "bgbv2 open safety":bool
  in  "cc3 open safety":bool
  in  "cc4 open safety":bool
  in  "cc1 open safety":bool
  in  "cc2 open safety":bool
  in  "tp3 start safety":bool
  in  "tp4 start safety":bool
  in  "tp2 start safety":bool
  in  "tp1 start safety":bool
  in  "plvbv4 open safety":bool
  in  "plvbv3 open safety":bool
  in  "plvbv1 open safety":bool
  in  "plvbv2 open safety":bool
  in  "chvbv4 open safety":bool
  in  "chvbv3 open safety":bool
  in  "chvbv1 open safety":bool
  in  "chvbv2 open safety":bool
  in  "tpbv1 close safety":bool
  in  "tpbv2 open safety":bool
  in  "tpbv1 open safety":bool
  in  "tpbv2 close safety":bool
  in  "tpbv3 open safety":bool
  in  "tpbv3 close safety":bool
  in  "tpbv4 open safety":bool
  in  "tpbv4 close safety":bool
  in  "mp1 stop safety":bool
  in  "mp2 start safety":bool
  in  "mp1 start safety":bool
  in  "mp2 stop safety":bool
  in  "mp3 start safety":bool
  in  "mp3 stop safety":bool
  in  "mp4 start safety":bool
  in  "mp4 stop safety":bool
  in  "ch1 trnsbp left open safety":bool
  in  "ch2 trnsbp right open safety":bool
  in  "ch2 trnsbp left open safety":bool
  in  "ch3 trnsbp right open safety":bool
  in  "ch3 trnsbp left open safety":bool
  in  "ch4 trnsbp right open safety":bool
  in  "CH1-2 trns open safety":bool
  in  "CH2-3 trns open safety":bool
  in  "CH3-4 trns open safety":bool
  in  "CH1-2 trns close safety":bool
  in  "CH2-3 trns close safety":bool
  in  "CH3-4 trns close safety":bool
  in  "CH2 safety cancel":bool
  in  "CH3 safety cancel":bool
  in  "CH4 safety cancel":bool
  in  "path to JPEG file":path=path "D:/VK-1701 System Files/Gui_new"
  out "Mouse Position":cluster{"X":i32, "Y":i32}
  out "Mouse .Button":bool
  out "resolution":dbl
  in  "Tp1 auto normal speed":bool
  in  "Tp1 auto low speed":bool
  in  "Tp1 auto set speed":bool
  in  "Tp1 auto stop":bool
  in  "Tp1 auto start":bool
  in  "Tp2 auto normal speed":bool
  in  "Tp2 auto low speed":bool
  in  "Tp2 auto set speed":bool
  in  "Tp2 auto stop":bool
  in  "Tp2 auto start":bool
  in  "Tp3 auto normal speed":bool
  in  "Tp3 auto low speed":bool